vi "generate and convert rnd 1,2,3-D arrays.vi"(0 "dims":i32, 1 "numeric type const":T1, 5 "Tag":string, 9 "sizes":T4, 11 "error in (no error)":errorcluster) -> (2 "current timepoint":dbl, 3 "Array 1D":cdb[](array[numeric]), 4 "Array 2D":cdb[][](array[numeric]), 6 "Array 3D":cdb[][][](array[numeric]), 8 "bytes":i32, 10 "array as variant":variant, 12 "element size (bytes)":u8, 13 "delta t (s)":dbl, 14 "Bindata & descr out":T2, 15 "error out":errorcluster)   [LabVIEW 2018, in "LV2Julia_examples.lvlib"]
uses:
  LV2Julia_examples.lvlib
  array 123D sizes.ctl
  LV2Julia_core/VIs/Bindata&description.ctl
  LV2Julia_core/VIs/Bindata description.ctl
  LV2Julia_core/VIs/Numeric Types enum.ctl
  85ae8d2b-1833-426f-a7e3-0aa59edb462e.vi
  b7a12c6c-f00d-43e6-9642-9243e32b2058.vi
  ba780daf-ef06-44ce-bff3-6c34795b2ca8.vi
  0827bc69-4216-4d70-a1a4-4bfc71e08fdd.vi
  31a52eb7-4f60-473e-a06e-05ec52e66b84.vi
  be087227-1c24-4c50-b280-a6b288463f93.vi
  1496614b-dcbf-47d4-84ca-bd6c1ad99fe0.vi
  1ec9265c-e1ac-4cb5-8500-03f8ca54a804.vi
  9cd03b83-d5bc-4a7f-9dd3-ef622f64ee30.vi
  ee83ef70-773d-469c-ba23-25239dc81b12.vi
  fca8e823-b190-45b9-9fbf-0f97a3b8de28.vi
  e5719774-7c0b-4606-b38f-adf2a3fe0ebf.vi
  0f763169-7436-48fd-a14e-d5e7c7a3701c.vi
  85ae8d2b-1833-426f-a7e3-0aa59edb462e.vi/c11693f3-b73f-4974-b2b1-4a09d7d4cdaa.vi
  85ae8d2b-1833-426f-a7e3-0aa59edb462e.vi/8e85eddd-eeb1-48c7-aa0c-acb2476f15c2.vi
  85ae8d2b-1833-426f-a7e3-0aa59edb462e.vi/23a185df-fff9-4986-ab04-d524cae2dab1.vi
  85ae8d2b-1833-426f-a7e3-0aa59edb462e.vi/111c06d2-3932-4e85-b4d7-53c92b5ae465.vi
  85ae8d2b-1833-426f-a7e3-0aa59edb462e.vi/af9a9771-594c-4ddf-b656-7825023e47e7.vi
  85ae8d2b-1833-426f-a7e3-0aa59edb462e.vi/a78b6e60-1a26-4501-a93d-f160922e020e.vi
  85ae8d2b-1833-426f-a7e3-0aa59edb462e.vi/f66aa46b-3816-4255-a4d3-c805dd2ce984.vi
  85ae8d2b-1833-426f-a7e3-0aa59edb462e.vi/619bb06e-8dfe-480d-80bb-ef92a1d4afee.vi
  85ae8d2b-1833-426f-a7e3-0aa59edb462e.vi/f9469cc9-c20f-42ad-af32-5d4df993a375.vi
  85ae8d2b-1833-426f-a7e3-0aa59edb462e.vi/711513a7-85bb-419e-9c32-aba576b50552.vi
  85ae8d2b-1833-426f-a7e3-0aa59edb462e.vi/823e16ca-39c9-487e-9eaf-1987967ec410.vi
  85ae8d2b-1833-426f-a7e3-0aa59edb462e.vi/5cb6cde2-b501-468b-ade4-7f718f27883f.vi
  85ae8d2b-1833-426f-a7e3-0aa59edb462e.vi/27d87cb8-d9ee-466a-8e4b-b166f897eca3.vi
  b7a12c6c-f00d-43e6-9642-9243e32b2058.vi/8f87c563-5639-42cc-9a08-28efbc45f0ff.vi
  b7a12c6c-f00d-43e6-9642-9243e32b2058.vi/0ada88ee-c4f2-4d17-bb7a-74a21d7765a4.vi
  b7a12c6c-f00d-43e6-9642-9243e32b2058.vi/11ebc9dc-4fee-49d4-b810-15b7504b15d2.vi
  b7a12c6c-f00d-43e6-9642-9243e32b2058.vi/3d2aaf23-1473-41e1-9c06-da7bddf8b942.vi
  b7a12c6c-f00d-43e6-9642-9243e32b2058.vi/502a5a5e-5782-46f9-888a-3583fb3fbf86.vi
  b7a12c6c-f00d-43e6-9642-9243e32b2058.vi/8f771d34-d398-4848-bcf1-8c49de59a304.vi
  b7a12c6c-f00d-43e6-9642-9243e32b2058.vi/a12f41f5-0570-4ac7-8c54-27b4d3e2bab2.vi
  b7a12c6c-f00d-43e6-9642-9243e32b2058.vi/4ef6f367-3f9b-4b1e-8355-75f10fbdbef3.vi
  b7a12c6c-f00d-43e6-9642-9243e32b2058.vi/963765af-ec1a-4af6-8576-dda3e1cb1b45.vi
  b7a12c6c-f00d-43e6-9642-9243e32b2058.vi/101da33c-8c0e-4aae-bc92-8a8eec4ebfb7.vi
  b7a12c6c-f00d-43e6-9642-9243e32b2058.vi/de32e5cb-40b1-4884-8d7d-a218bab2078b.vi
  b7a12c6c-f00d-43e6-9642-9243e32b2058.vi/07cbf523-cf59-4f94-853d-da613bdf1b42.vi
  b7a12c6c-f00d-43e6-9642-9243e32b2058.vi/b7acff62-395d-4c96-ac40-70f2153a0cea.vi
  ba780daf-ef06-44ce-bff3-6c34795b2ca8.vi/3d2c9a32-9bf9-4bce-8a47-0e79a702d242.vi
  ba780daf-ef06-44ce-bff3-6c34795b2ca8.vi/faf0b0c0-115a-4e37-90b8-e50dcc4168bc.vi
  ba780daf-ef06-44ce-bff3-6c34795b2ca8.vi/94a6b6ae-9615-428f-8d56-76a1308c1a35.vi
  ba780daf-ef06-44ce-bff3-6c34795b2ca8.vi/534bd078-003c-4e2f-ad5e-8e7ac9c68b32.vi
  ba780daf-ef06-44ce-bff3-6c34795b2ca8.vi/3ee41887-da2e-4051-ad5a-82b4c75e16db.vi
  ba780daf-ef06-44ce-bff3-6c34795b2ca8.vi/67149314-f5ff-427e-8ec6-2ec35dc5d17a.vi
  ba780daf-ef06-44ce-bff3-6c34795b2ca8.vi/7898d58a-5049-4ff7-961b-0aadd4609598.vi
  ba780daf-ef06-44ce-bff3-6c34795b2ca8.vi/85423b60-0515-46bc-807a-fbd470e65e28.vi
  ba780daf-ef06-44ce-bff3-6c34795b2ca8.vi/440f1969-f94a-49e7-92dd-969720926e87.vi
  ba780daf-ef06-44ce-bff3-6c34795b2ca8.vi/2286e7bd-8b3c-4844-af13-d0199e238791.vi
  ba780daf-ef06-44ce-bff3-6c34795b2ca8.vi/3ef977eb-8b9d-4e48-9cda-ed62cb7b638c.vi
  ba780daf-ef06-44ce-bff3-6c34795b2ca8.vi/10ae00de-f8c8-4d89-829e-497fdc340f77.vi
  ba780daf-ef06-44ce-bff3-6c34795b2ca8.vi/da656cc8-e788-4d5a-baa0-4a07c0a2dc57.vi
  0827bc69-4216-4d70-a1a4-4bfc71e08fdd.vi/0ffb3e9e-3e66-4f14-a53f-c9719ec25faa.vi
  0827bc69-4216-4d70-a1a4-4bfc71e08fdd.vi/261e91eb-d6ba-4368-8adb-b056b6d5af16.vi
  0827bc69-4216-4d70-a1a4-4bfc71e08fdd.vi/9ea1f025-802d-4756-ba0d-f9222c4a6e71.vi
  0827bc69-4216-4d70-a1a4-4bfc71e08fdd.vi/ce551d52-1534-428d-b95b-163587a632ea.vi
  0827bc69-4216-4d70-a1a4-4bfc71e08fdd.vi/1cb40332-89ee-4e85-bdd1-f055d6e9593b.vi
  0827bc69-4216-4d70-a1a4-4bfc71e08fdd.vi/6f9467ea-fd04-4604-ae84-ffea5ad4eb15.vi
  0827bc69-4216-4d70-a1a4-4bfc71e08fdd.vi/8b14cc06-0996-4e9e-9771-b4637b9f2da9.vi
  0827bc69-4216-4d70-a1a4-4bfc71e08fdd.vi/2aac3158-face-4bd6-b9ad-b375428daa75.vi
  0827bc69-4216-4d70-a1a4-4bfc71e08fdd.vi/dca4cbc9-ee5f-4956-bc16-6b9268f2ae46.vi
  0827bc69-4216-4d70-a1a4-4bfc71e08fdd.vi/0304a7fd-9da4-4c9e-b22c-ccf287610983.vi
  31a52eb7-4f60-473e-a06e-05ec52e66b84.vi/8cb8b6d6-c350-4b2b-a0a8-0d2690d8b07b.vi
  31a52eb7-4f60-473e-a06e-05ec52e66b84.vi/833f7a80-f94e-40d2-8863-3d22036f4c05.vi
  31a52eb7-4f60-473e-a06e-05ec52e66b84.vi/d31a9b35-cfb5-4c2d-966c-d447f74259d9.vi
  31a52eb7-4f60-473e-a06e-05ec52e66b84.vi/accceabc-846c-4be5-962f-1824ae5aaede.vi
  31a52eb7-4f60-473e-a06e-05ec52e66b84.vi/4dc64207-d105-4bdf-b337-3f5f3ae1db54.vi
  31a52eb7-4f60-473e-a06e-05ec52e66b84.vi/62b8defa-d172-4f34-a887-d316d84189de.vi
  31a52eb7-4f60-473e-a06e-05ec52e66b84.vi/9afc9c51-9b27-4e76-89bd-75c50f9c723a.vi
  31a52eb7-4f60-473e-a06e-05ec52e66b84.vi/bd806f5f-2604-4275-b291-1a75ab4434d2.vi
  31a52eb7-4f60-473e-a06e-05ec52e66b84.vi/caebaab9-5afa-4ebd-88ee-492fb4ee9da6.vi
  31a52eb7-4f60-473e-a06e-05ec52e66b84.vi/e039d2d0-3bbc-4582-81ec-187b9517587b.vi
  31a52eb7-4f60-473e-a06e-05ec52e66b84.vi/9568bcd8-1bcd-454b-a48d-3b86cd522847.vi
  31a52eb7-4f60-473e-a06e-05ec52e66b84.vi/09ab5422-ef20-4763-a888-a938fed40b0e.vi
  31a52eb7-4f60-473e-a06e-05ec52e66b84.vi/2e676773-8913-4cea-aabf-fdbe2542e0f5.vi
  be087227-1c24-4c50-b280-a6b288463f93.vi/e0bc1a08-e00b-451c-b5ab-4c6982896503.vi
  be087227-1c24-4c50-b280-a6b288463f93.vi/77d648b1-c2bd-47e8-9d98-d5979e8947bd.vi
  be087227-1c24-4c50-b280-a6b288463f93.vi/65d82d02-bd24-4674-9173-3ed41e56919b.vi
  be087227-1c24-4c50-b280-a6b288463f93.vi/18b04783-ed4b-4ee5-89ff-fd61c120f221.vi
  be087227-1c24-4c50-b280-a6b288463f93.vi/9db986cd-cad9-4629-9f04-d611e563b09c.vi
  be087227-1c24-4c50-b280-a6b288463f93.vi/f6b59062-e60a-42fa-ac54-cd6239ac50ba.vi
  be087227-1c24-4c50-b280-a6b288463f93.vi/d2924102-86a5-4d3f-871d-219b5fa01cfc.vi
  be087227-1c24-4c50-b280-a6b288463f93.vi/32bc084b-fb97-4fe6-aed2-634cc9ae6959.vi
  be087227-1c24-4c50-b280-a6b288463f93.vi/67544f08-8803-4e76-831f-e149eee3dcfb.vi
  be087227-1c24-4c50-b280-a6b288463f93.vi/f21d593f-3e97-4790-a451-2b207607bde3.vi
  be087227-1c24-4c50-b280-a6b288463f93.vi/ea729439-b51a-49c6-8548-a99ef89a8bee.vi
  be087227-1c24-4c50-b280-a6b288463f93.vi/031cee27-362f-4823-977f-ed077a2a16a0.vi
  be087227-1c24-4c50-b280-a6b288463f93.vi/c69ce045-6d3b-444d-827b-39663dd71d37.vi
  1496614b-dcbf-47d4-84ca-bd6c1ad99fe0.vi/c01cb2f5-b56f-414d-9efa-4711ccf5838c.vi
  1496614b-dcbf-47d4-84ca-bd6c1ad99fe0.vi/47715fe6-eadc-4bbe-9722-e67c6229c693.vi
  1496614b-dcbf-47d4-84ca-bd6c1ad99fe0.vi/467e9573-caa5-4b84-adeb-55ebcd8aef26.vi
  1496614b-dcbf-47d4-84ca-bd6c1ad99fe0.vi/62ca9728-5259-4073-b318-c3e87ac254fb.vi
  1496614b-dcbf-47d4-84ca-bd6c1ad99fe0.vi/8a8a2384-441c-4f35-bc10-b3d32a1405b6.vi
  1496614b-dcbf-47d4-84ca-bd6c1ad99fe0.vi/521b95e9-0149-4117-abe1-2fb16e8ae733.vi
  1496614b-dcbf-47d4-84ca-bd6c1ad99fe0.vi/df480a62-78f0-42ce-87d6-259297a748c5.vi
  1496614b-dcbf-47d4-84ca-bd6c1ad99fe0.vi/9c38cd94-90ac-4a24-bfaa-0db9f25f4733.vi
  1496614b-dcbf-47d4-84ca-bd6c1ad99fe0.vi/a5d379dd-b135-4ded-bacd-aaa1ef77f126.vi
  1496614b-dcbf-47d4-84ca-bd6c1ad99fe0.vi/ccc82a22-f0d8-46b3-875d-cd0015cd561e.vi
  1496614b-dcbf-47d4-84ca-bd6c1ad99fe0.vi/9c5b4bee-1a68-423a-91f1-797d0648e215.vi
  1496614b-dcbf-47d4-84ca-bd6c1ad99fe0.vi/6666430c-a415-47dd-a618-32a1bea4c343.vi
  1496614b-dcbf-47d4-84ca-bd6c1ad99fe0.vi/3ff0d97e-381d-4f66-8109-0f3fcc348163.vi
  1ec9265c-e1ac-4cb5-8500-03f8ca54a804.vi/7b0e696b-714e-4af6-aa69-c94e202e048f.vi
  1ec9265c-e1ac-4cb5-8500-03f8ca54a804.vi/ab8334bc-80fe-49a7-aeaa-72d4d4d986e9.vi
  1ec9265c-e1ac-4cb5-8500-03f8ca54a804.vi/0ffb9047-8700-4382-b3d0-3373f475b523.vi
  1ec9265c-e1ac-4cb5-8500-03f8ca54a804.vi/d0489657-9c20-4211-801e-dddad1e2d8d8.vi
  1ec9265c-e1ac-4cb5-8500-03f8ca54a804.vi/96353e94-dd23-4035-8dd4-90333fc8a4d3.vi
  1ec9265c-e1ac-4cb5-8500-03f8ca54a804.vi/bcc4aa1a-f580-4222-a6ed-dc128524a11c.vi
  1ec9265c-e1ac-4cb5-8500-03f8ca54a804.vi/a02a3a82-3c87-4f5a-bd2d-74660287815d.vi
  1ec9265c-e1ac-4cb5-8500-03f8ca54a804.vi/cb715031-fb8a-4382-9ede-7ffb25dbcc6b.vi
  1ec9265c-e1ac-4cb5-8500-03f8ca54a804.vi/167585a2-6b26-4dd4-a205-ebd7312b44a1.vi
  1ec9265c-e1ac-4cb5-8500-03f8ca54a804.vi/c12c282e-0894-4e11-9b84-b0275f3ed5c5.vi
  1ec9265c-e1ac-4cb5-8500-03f8ca54a804.vi/645016e3-e720-4573-9a54-e364668f4a88.vi
  1ec9265c-e1ac-4cb5-8500-03f8ca54a804.vi/c54be713-0bde-4142-a465-061db3609d3a.vi
  1ec9265c-e1ac-4cb5-8500-03f8ca54a804.vi/35d82dd1-5997-4dad-a75b-413ba1ea936f.vi
  9cd03b83-d5bc-4a7f-9dd3-ef622f64ee30.vi/93e2137a-2cb5-4f0c-ad93-c6e9d1e8eedd.vi
  9cd03b83-d5bc-4a7f-9dd3-ef622f64ee30.vi/c26303ed-4f99-4591-9769-7eebad8d47fd.vi
  9cd03b83-d5bc-4a7f-9dd3-ef622f64ee30.vi/9d67a838-50a0-44f0-824e-bcc4b1f4de21.vi
  9cd03b83-d5bc-4a7f-9dd3-ef622f64ee30.vi/ee5e38f0-2884-47d9-890d-5561dd5d35b6.vi
  9cd03b83-d5bc-4a7f-9dd3-ef622f64ee30.vi/401e3ff0-0d76-40e6-a2f4-d101c51ec70e.vi
  9cd03b83-d5bc-4a7f-9dd3-ef622f64ee30.vi/96e80ebc-e1b5-4129-8640-c2de42f87428.vi
  9cd03b83-d5bc-4a7f-9dd3-ef622f64ee30.vi/e4cfc389-a6ad-47a7-8c7b-2ea402abe593.vi
  9cd03b83-d5bc-4a7f-9dd3-ef622f64ee30.vi/28e1bac3-2967-4b4f-8496-3cdb4949f6da.vi
  9cd03b83-d5bc-4a7f-9dd3-ef622f64ee30.vi/b4056afe-3c0d-4dbc-a3cd-b11ce2b05076.vi
  9cd03b83-d5bc-4a7f-9dd3-ef622f64ee30.vi/b774ffbc-34c7-43f5-abf3-881f626a4619.vi
  9cd03b83-d5bc-4a7f-9dd3-ef622f64ee30.vi/61b4febb-0523-454e-81e2-ddeff6ec8b17.vi
  9cd03b83-d5bc-4a7f-9dd3-ef622f64ee30.vi/b4698ce2-e08e-4695-94f2-7ed1591759de.vi
  9cd03b83-d5bc-4a7f-9dd3-ef622f64ee30.vi/a27f1cb3-c6ce-4ccd-a6a6-1e7befeb3bd1.vi
  ee83ef70-773d-469c-ba23-25239dc81b12.vi/b6b2f408-bd09-4a05-87e2-6bb6c3fd5077.vi
  ee83ef70-773d-469c-ba23-25239dc81b12.vi/c87a68b0-2172-4a67-a6f0-f210c7451bd3.vi
  ee83ef70-773d-469c-ba23-25239dc81b12.vi/6c78d6e0-c22e-4947-a458-bffffac5c58a.vi
  ee83ef70-773d-469c-ba23-25239dc81b12.vi/5de9532b-c5af-408b-877c-e74a5a4f0c58.vi
  ee83ef70-773d-469c-ba23-25239dc81b12.vi/4135ce50-1702-49d5-b7b5-9d498c87c660.vi
  ee83ef70-773d-469c-ba23-25239dc81b12.vi/12f1fc26-1317-442f-838f-3b2e5da797d4.vi
  ee83ef70-773d-469c-ba23-25239dc81b12.vi/a37e5f57-4ce8-4f63-824f-30bd9374e42d.vi
  ee83ef70-773d-469c-ba23-25239dc81b12.vi/9c434990-2cfd-4912-9f2b-e35b427005c7.vi
  ee83ef70-773d-469c-ba23-25239dc81b12.vi/9914fa42-08c7-43b8-a27e-b62889b56e78.vi
  ee83ef70-773d-469c-ba23-25239dc81b12.vi/12eed14b-2360-4d7b-a8c7-2760bfb367f4.vi
  ee83ef70-773d-469c-ba23-25239dc81b12.vi/36fb79f1-b7e4-4398-a5d0-b20316fc2697.vi
  ee83ef70-773d-469c-ba23-25239dc81b12.vi/2274937d-171b-46e1-8bea-50482967b9d6.vi
  ee83ef70-773d-469c-ba23-25239dc81b12.vi/f37db113-05b9-42a2-9ee4-f62b43b889a4.vi
  fca8e823-b190-45b9-9fbf-0f97a3b8de28.vi/a7974878-4d5e-4b05-880b-0f64ae5ea67a.vi
  fca8e823-b190-45b9-9fbf-0f97a3b8de28.vi/a46cdcc9-52d0-4030-83dd-4ce08d19186e.vi
  fca8e823-b190-45b9-9fbf-0f97a3b8de28.vi/3059a3e2-810f-488e-a970-9e32afe7d42e.vi
  fca8e823-b190-45b9-9fbf-0f97a3b8de28.vi/6f505528-69ad-402a-8405-961601b8f439.vi
  fca8e823-b190-45b9-9fbf-0f97a3b8de28.vi/4dbc5799-ec76-42b3-bb12-e906c396b96b.vi
  fca8e823-b190-45b9-9fbf-0f97a3b8de28.vi/b67824c8-14c1-498a-a365-be7e5b9e05a9.vi
  fca8e823-b190-45b9-9fbf-0f97a3b8de28.vi/3cc7adc6-ea27-40fe-a2af-02b14d132bf1.vi
  fca8e823-b190-45b9-9fbf-0f97a3b8de28.vi/6f9b27ce-9f3e-402d-ab85-ab46fe6c97b8.vi
  fca8e823-b190-45b9-9fbf-0f97a3b8de28.vi/cb420030-84f1-4efb-80b2-f5620303c743.vi
  fca8e823-b190-45b9-9fbf-0f97a3b8de28.vi/6eb4f9ed-08d2-487c-a94c-fc4702305324.vi
  fca8e823-b190-45b9-9fbf-0f97a3b8de28.vi/8760845b-1db7-4683-9605-4adb35927513.vi
  fca8e823-b190-45b9-9fbf-0f97a3b8de28.vi/31762919-4fdd-4e4e-9867-659220ffc92a.vi
  fca8e823-b190-45b9-9fbf-0f97a3b8de28.vi/66a9a665-6ada-42a7-a9ee-cefd3614f9db.vi
  e5719774-7c0b-4606-b38f-adf2a3fe0ebf.vi/cb8d9f8b-f77d-441c-9a50-6a25f90cdb3a.vi
  e5719774-7c0b-4606-b38f-adf2a3fe0ebf.vi/e04a025a-b044-48ec-9ce3-537d6650ec9f.vi
  e5719774-7c0b-4606-b38f-adf2a3fe0ebf.vi/55e2d376-65fc-4653-9a58-b62012819d29.vi
  e5719774-7c0b-4606-b38f-adf2a3fe0ebf.vi/6dcd6532-d588-4e67-872e-414ffbc19b0e.vi
  e5719774-7c0b-4606-b38f-adf2a3fe0ebf.vi/6399dd36-c1e6-41ee-ae47-d998c15f331f.vi
  e5719774-7c0b-4606-b38f-adf2a3fe0ebf.vi/2a064c1c-8aca-47db-8768-36cf0793d53c.vi
  e5719774-7c0b-4606-b38f-adf2a3fe0ebf.vi/6f8860ea-d4c0-4767-a922-dedba0ba4007.vi
  e5719774-7c0b-4606-b38f-adf2a3fe0ebf.vi/b041bd99-f132-49ce-8946-2be68e4cf2ac.vi
  e5719774-7c0b-4606-b38f-adf2a3fe0ebf.vi/c5e050e8-c7cb-4905-8055-5f2d77b4ebae.vi
  e5719774-7c0b-4606-b38f-adf2a3fe0ebf.vi/7ed19e76-0a08-47ca-b695-626adb0ec6f7.vi
  e5719774-7c0b-4606-b38f-adf2a3fe0ebf.vi/d7daec0d-9f20-43c2-b0bb-c95e8d390d79.vi
  e5719774-7c0b-4606-b38f-adf2a3fe0ebf.vi/9222370a-7fee-43cb-90a9-f0df0c454ece.vi
  e5719774-7c0b-4606-b38f-adf2a3fe0ebf.vi/b53ecc98-60f0-47c7-b08c-58bd9e3a996b.vi
  0f763169-7436-48fd-a14e-d5e7c7a3701c.vi/045392a4-ec50-4749-8bf5-54c1fbda4d0b.vi
  0f763169-7436-48fd-a14e-d5e7c7a3701c.vi/4318b9fa-7e96-4320-ad14-e58bf08cbdca.vi
  0f763169-7436-48fd-a14e-d5e7c7a3701c.vi/cfbc86c3-8a1d-4456-a249-fc06cd6d8936.vi
  0f763169-7436-48fd-a14e-d5e7c7a3701c.vi/72299fb9-025a-424e-bf32-5f05b2a8e981.vi
  0f763169-7436-48fd-a14e-d5e7c7a3701c.vi/42337aaa-b56a-45f8-8fc1-26a400602ff7.vi
  0f763169-7436-48fd-a14e-d5e7c7a3701c.vi/04b2a31c-4aaa-4239-a820-f2446d749457.vi
  0f763169-7436-48fd-a14e-d5e7c7a3701c.vi/64641c69-3eb6-4d25-a9bc-e555532b6975.vi
  0f763169-7436-48fd-a14e-d5e7c7a3701c.vi/ff7bb5cf-0953-422c-b9dd-7e5e3a8e3007.vi
  0f763169-7436-48fd-a14e-d5e7c7a3701c.vi/6ec92a7e-3200-4835-a3af-72f6deb2a7de.vi
  0f763169-7436-48fd-a14e-d5e7c7a3701c.vi/3914dbf0-1a68-4dc6-be7c-ff95f1d0b2d4.vi
  0f763169-7436-48fd-a14e-d5e7c7a3701c.vi/b66477fe-308b-4a84-8565-e124399292a6.vi
  0f763169-7436-48fd-a14e-d5e7c7a3701c.vi/e46fa793-5279-4872-b6f8-63be130737c1.vi
  0f763169-7436-48fd-a14e-d5e7c7a3701c.vi/52a5156d-4e95-4ff6-b9e4-83278f7f7ef3.vi
  85ae8d2b-1833-426f-a7e3-0aa59edb462e.vi/8e85eddd-eeb1-48c7-aa0c-acb2476f15c2.vi/08ea7271-58f7-4381-bb13-89612bf68987.vi
  <vilib>/Utility/High Resolution Relative Seconds.vi
  85ae8d2b-1833-426f-a7e3-0aa59edb462e.vi/af9a9771-594c-4ddf-b656-7825023e47e7.vi/a558cd4b-dbd0-4514-827e-24ca6e6b3a91.vi
  85ae8d2b-1833-426f-a7e3-0aa59edb462e.vi/f9469cc9-c20f-42ad-af32-5d4df993a375.vi/8c409728-000f-45f8-9ccd-ee15c7ed8521.vi
  b7a12c6c-f00d-43e6-9642-9243e32b2058.vi/0ada88ee-c4f2-4d17-bb7a-74a21d7765a4.vi/69bbc40a-c36a-4917-aaee-edada7b7b8d7.vi
  b7a12c6c-f00d-43e6-9642-9243e32b2058.vi/502a5a5e-5782-46f9-888a-3583fb3fbf86.vi/571e470d-9707-4b89-9631-5b8d9304f753.vi
  b7a12c6c-f00d-43e6-9642-9243e32b2058.vi/963765af-ec1a-4af6-8576-dda3e1cb1b45.vi/a9e7bee4-94d8-4d8e-b190-a2971037c66e.vi
  ba780daf-ef06-44ce-bff3-6c34795b2ca8.vi/faf0b0c0-115a-4e37-90b8-e50dcc4168bc.vi/ff37c594-a005-47f5-bb34-4c70a0126acb.vi
  ba780daf-ef06-44ce-bff3-6c34795b2ca8.vi/3ee41887-da2e-4051-ad5a-82b4c75e16db.vi/43312af0-9a58-49ee-9340-b8aa225bd272.vi
  ba780daf-ef06-44ce-bff3-6c34795b2ca8.vi/440f1969-f94a-49e7-92dd-969720926e87.vi/1b453ea8-962a-4255-a994-0cbca27764d4.vi
  0827bc69-4216-4d70-a1a4-4bfc71e08fdd.vi/261e91eb-d6ba-4368-8adb-b056b6d5af16.vi/d1f6d98c-0505-4e61-9b8c-a3eed1ff26ed.vi
  0827bc69-4216-4d70-a1a4-4bfc71e08fdd.vi/1cb40332-89ee-4e85-bdd1-f055d6e9593b.vi/3667db32-83c2-4485-8485-501a99b88cfe.vi
  0827bc69-4216-4d70-a1a4-4bfc71e08fdd.vi/2aac3158-face-4bd6-b9ad-b375428daa75.vi/10b5fca0-4c2a-4c9a-8b53-fb3dcff5ab00.vi
  31a52eb7-4f60-473e-a06e-05ec52e66b84.vi/833f7a80-f94e-40d2-8863-3d22036f4c05.vi/de0d82be-3b4d-4b69-b774-1ee66ef3b500.vi
  31a52eb7-4f60-473e-a06e-05ec52e66b84.vi/4dc64207-d105-4bdf-b337-3f5f3ae1db54.vi/7b76e6e9-99fc-48fe-88e5-663e33f1532b.vi
  31a52eb7-4f60-473e-a06e-05ec52e66b84.vi/caebaab9-5afa-4ebd-88ee-492fb4ee9da6.vi/ae77f17b-7a63-49d8-8677-2eb378eecda7.vi
  be087227-1c24-4c50-b280-a6b288463f93.vi/77d648b1-c2bd-47e8-9d98-d5979e8947bd.vi/eb2ac645-ddc7-47bc-9d8b-75952129f04e.vi
  be087227-1c24-4c50-b280-a6b288463f93.vi/9db986cd-cad9-4629-9f04-d611e563b09c.vi/b1da1a18-7165-4dcd-a4ff-b5fd07c18a7e.vi
  be087227-1c24-4c50-b280-a6b288463f93.vi/67544f08-8803-4e76-831f-e149eee3dcfb.vi/541c202c-62e7-4b26-a949-153a4b69c346.vi
  1496614b-dcbf-47d4-84ca-bd6c1ad99fe0.vi/47715fe6-eadc-4bbe-9722-e67c6229c693.vi/0fdc2738-6627-4de2-9d66-c6113426bbea.vi
  1496614b-dcbf-47d4-84ca-bd6c1ad99fe0.vi/8a8a2384-441c-4f35-bc10-b3d32a1405b6.vi/9880d032-961f-4e8d-bd85-807a3cb9978c.vi
  1496614b-dcbf-47d4-84ca-bd6c1ad99fe0.vi/a5d379dd-b135-4ded-bacd-aaa1ef77f126.vi/d1569549-6e2f-4408-83e1-6f356c70d908.vi
  1ec9265c-e1ac-4cb5-8500-03f8ca54a804.vi/ab8334bc-80fe-49a7-aeaa-72d4d4d986e9.vi/b9ff3e0a-05c7-4d11-a75b-368fec092445.vi
  1ec9265c-e1ac-4cb5-8500-03f8ca54a804.vi/96353e94-dd23-4035-8dd4-90333fc8a4d3.vi/f4ce16f9-675e-447e-8c5f-32c7ef14206e.vi
  1ec9265c-e1ac-4cb5-8500-03f8ca54a804.vi/167585a2-6b26-4dd4-a205-ebd7312b44a1.vi/4f7bf506-ab24-41ce-b71a-8160a5476407.vi
  9cd03b83-d5bc-4a7f-9dd3-ef622f64ee30.vi/c26303ed-4f99-4591-9769-7eebad8d47fd.vi/1b763a9f-5ce5-41ba-bc7f-9f995f4d2b4d.vi
  9cd03b83-d5bc-4a7f-9dd3-ef622f64ee30.vi/401e3ff0-0d76-40e6-a2f4-d101c51ec70e.vi/66e2e3b0-dc28-4f05-a834-250e6508c857.vi
  9cd03b83-d5bc-4a7f-9dd3-ef622f64ee30.vi/b4056afe-3c0d-4dbc-a3cd-b11ce2b05076.vi/40f3e5bb-f60e-451c-8b00-4309ab568451.vi
  ee83ef70-773d-469c-ba23-25239dc81b12.vi/c87a68b0-2172-4a67-a6f0-f210c7451bd3.vi/84a80026-1c80-486c-8d92-8831a7df5ff3.vi
  ee83ef70-773d-469c-ba23-25239dc81b12.vi/4135ce50-1702-49d5-b7b5-9d498c87c660.vi/d1bc0e7f-a379-4ff9-bf17-9e41a0f46a57.vi
  ee83ef70-773d-469c-ba23-25239dc81b12.vi/9914fa42-08c7-43b8-a27e-b62889b56e78.vi/5de439e2-5012-4648-894c-bb1b9ad5bb26.vi
  fca8e823-b190-45b9-9fbf-0f97a3b8de28.vi/a46cdcc9-52d0-4030-83dd-4ce08d19186e.vi/90bccda5-6ac7-4d46-9afb-e6399bdb2e1f.vi
  fca8e823-b190-45b9-9fbf-0f97a3b8de28.vi/4dbc5799-ec76-42b3-bb12-e906c396b96b.vi/ec007a79-76e9-41e5-8892-0302a9e6b40b.vi
  fca8e823-b190-45b9-9fbf-0f97a3b8de28.vi/cb420030-84f1-4efb-80b2-f5620303c743.vi/2c209796-9244-4d59-a9f5-eb5b4e6512ff.vi
  e5719774-7c0b-4606-b38f-adf2a3fe0ebf.vi/e04a025a-b044-48ec-9ce3-537d6650ec9f.vi/be8c913f-5955-4425-929d-934409af2b49.vi
  e5719774-7c0b-4606-b38f-adf2a3fe0ebf.vi/6399dd36-c1e6-41ee-ae47-d998c15f331f.vi/49d2f734-92bf-43e0-a325-d114aa2d52b5.vi
  e5719774-7c0b-4606-b38f-adf2a3fe0ebf.vi/c5e050e8-c7cb-4905-8055-5f2d77b4ebae.vi/22426407-5a39-4ae1-b419-51b886c4e6cc.vi
  0f763169-7436-48fd-a14e-d5e7c7a3701c.vi/4318b9fa-7e96-4320-ad14-e58bf08cbdca.vi/ec80edef-ad4d-481c-bae0-ad236ad91d17.vi
  0f763169-7436-48fd-a14e-d5e7c7a3701c.vi/42337aaa-b56a-45f8-8fc1-26a400602ff7.vi/853c4e43-66a7-4fd6-8a67-725115d20b02.vi
  0f763169-7436-48fd-a14e-d5e7c7a3701c.vi/6ec92a7e-3200-4835-a3af-72f6deb2a7de.vi/d7fa0239-54ab-48c8-b35d-0719727c3c46.vi
  85ae8d2b-1833-426f-a7e3-0aa59edb462e.vi/8e85eddd-eeb1-48c7-aa0c-acb2476f15c2.vi/08ea7271-58f7-4381-bb13-89612bf68987.vi/c319c975-6598-4c49-9112-e1ac8bec7b87.vi
  85ae8d2b-1833-426f-a7e3-0aa59edb462e.vi/af9a9771-594c-4ddf-b656-7825023e47e7.vi/a558cd4b-dbd0-4514-827e-24ca6e6b3a91.vi/23666670-5fa0-4551-929a-5078f8c88eb4.vi
  85ae8d2b-1833-426f-a7e3-0aa59edb462e.vi/f9469cc9-c20f-42ad-af32-5d4df993a375.vi/8c409728-000f-45f8-9ccd-ee15c7ed8521.vi/af52c658-7aca-4654-a19b-bdc00d5bce4f.vi
  b7a12c6c-f00d-43e6-9642-9243e32b2058.vi/0ada88ee-c4f2-4d17-bb7a-74a21d7765a4.vi/69bbc40a-c36a-4917-aaee-edada7b7b8d7.vi/c11b2df1-177a-40a7-9ba6-98232f8d7f99.vi
  b7a12c6c-f00d-43e6-9642-9243e32b2058.vi/502a5a5e-5782-46f9-888a-3583fb3fbf86.vi/571e470d-9707-4b89-9631-5b8d9304f753.vi/e1749920-efd2-42e0-885b-7fb6c4c5ab43.vi
  b7a12c6c-f00d-43e6-9642-9243e32b2058.vi/963765af-ec1a-4af6-8576-dda3e1cb1b45.vi/a9e7bee4-94d8-4d8e-b190-a2971037c66e.vi/1f67fc8e-8653-4e8b-a6c2-2cf9980ddd08.vi
  ba780daf-ef06-44ce-bff3-6c34795b2ca8.vi/faf0b0c0-115a-4e37-90b8-e50dcc4168bc.vi/ff37c594-a005-47f5-bb34-4c70a0126acb.vi/c6e85278-50f0-4f6a-9193-dc1bcd0ef70f.vi
  ba780daf-ef06-44ce-bff3-6c34795b2ca8.vi/3ee41887-da2e-4051-ad5a-82b4c75e16db.vi/43312af0-9a58-49ee-9340-b8aa225bd272.vi/3269ca27-2cba-45df-9346-92c5d96bd6fc.vi
  ba780daf-ef06-44ce-bff3-6c34795b2ca8.vi/440f1969-f94a-49e7-92dd-969720926e87.vi/1b453ea8-962a-4255-a994-0cbca27764d4.vi/f62144a5-f5db-4e00-a07d-a8ab4245d2e0.vi
  0827bc69-4216-4d70-a1a4-4bfc71e08fdd.vi/261e91eb-d6ba-4368-8adb-b056b6d5af16.vi/d1f6d98c-0505-4e61-9b8c-a3eed1ff26ed.vi/7d30ac35-157d-4fcc-9b6f-176c22041dd3.vi
  0827bc69-4216-4d70-a1a4-4bfc71e08fdd.vi/1cb40332-89ee-4e85-bdd1-f055d6e9593b.vi/3667db32-83c2-4485-8485-501a99b88cfe.vi/a5ed325d-485e-44f9-b4a5-b94842094a7d.vi
  0827bc69-4216-4d70-a1a4-4bfc71e08fdd.vi/2aac3158-face-4bd6-b9ad-b375428daa75.vi/10b5fca0-4c2a-4c9a-8b53-fb3dcff5ab00.vi/83375121-0e11-44d4-aa51-0de5076e5d92.vi
  31a52eb7-4f60-473e-a06e-05ec52e66b84.vi/833f7a80-f94e-40d2-8863-3d22036f4c05.vi/de0d82be-3b4d-4b69-b774-1ee66ef3b500.vi/3a45cae5-de8a-427f-805d-7805f64916c3.vi
  31a52eb7-4f60-473e-a06e-05ec52e66b84.vi/4dc64207-d105-4bdf-b337-3f5f3ae1db54.vi/7b76e6e9-99fc-48fe-88e5-663e33f1532b.vi/06f57519-d6ad-4a96-9600-46d432553020.vi
  31a52eb7-4f60-473e-a06e-05ec52e66b84.vi/caebaab9-5afa-4ebd-88ee-492fb4ee9da6.vi/ae77f17b-7a63-49d8-8677-2eb378eecda7.vi/07361902-21c8-49bd-b0fa-bce76e827913.vi
  be087227-1c24-4c50-b280-a6b288463f93.vi/77d648b1-c2bd-47e8-9d98-d5979e8947bd.vi/eb2ac645-ddc7-47bc-9d8b-75952129f04e.vi/90e6bd1a-94b1-4e35-a711-208e6fb95ce0.vi
  be087227-1c24-4c50-b280-a6b288463f93.vi/9db986cd-cad9-4629-9f04-d611e563b09c.vi/b1da1a18-7165-4dcd-a4ff-b5fd07c18a7e.vi/e9ab5a05-9916-45bc-bc4c-428d98bb0cc0.vi
  be087227-1c24-4c50-b280-a6b288463f93.vi/67544f08-8803-4e76-831f-e149eee3dcfb.vi/541c202c-62e7-4b26-a949-153a4b69c346.vi/04e1edd0-f714-4231-8a6f-30cd0f5f9b80.vi
  1496614b-dcbf-47d4-84ca-bd6c1ad99fe0.vi/47715fe6-eadc-4bbe-9722-e67c6229c693.vi/0fdc2738-6627-4de2-9d66-c6113426bbea.vi/30918f85-42e6-4e48-8a75-a92bfcdedf97.vi
  1496614b-dcbf-47d4-84ca-bd6c1ad99fe0.vi/8a8a2384-441c-4f35-bc10-b3d32a1405b6.vi/9880d032-961f-4e8d-bd85-807a3cb9978c.vi/30cf2ff2-8458-4241-b44f-73b870a3098c.vi
  1496614b-dcbf-47d4-84ca-bd6c1ad99fe0.vi/a5d379dd-b135-4ded-bacd-aaa1ef77f126.vi/d1569549-6e2f-4408-83e1-6f356c70d908.vi/aa36f776-024c-45ea-9348-02a91e581604.vi